vi "Super Market Billing System Edited.vi"() -> ()   [LabVIEW 2021]
uses:
  <vilib>/Utility/file.llb/Write Delimited Spreadsheet (string).vi
  <vilib>/regexp/Match Regular Expression.xnode
panel:
  in  "Tab Control":enum32{"Page 1", "Page 2", "Page 3"}(tab)
  out "Horizontal Progress Bar":u8(slide) scale=0.0..100.0
  in  "Password":string
  in  "Cashier User Name":string
  in  "OK Button":bool
  in  "Rise 5Kg":bool
  in  "Dal 1Kg":bool
  in  "Salt 400g":bool
  in  "Coconut Oil 1L":bool
  in  "Cilli Powder 100g":bool
  in  "Curry Powder 100g":bool
  in  "Turmeric Powder 50g":bool
  in  "Milk Powder 1kg":bool
  in  "Sugar  1kg":bool
  out "Rs.":dbl
  out "Rs.":dbl
  out "Rs.":dbl
  out "Rs.":dbl
  in  "Quantitiy":dbl min=0.0 format="%#.1f"
  out "Rs.":dbl
  in  "Quantitiy":dbl min=0.0 format="%#.1f"
  out "Rs":dbl
  in  "Quantitiy":dbl min=0.0 format="%#.1f"
  out "Rs.":dbl
  in  "Quantitiy":dbl min=0.0 format="%#.1f"
  in  "Quantitiy":dbl min=0.0 format="%#.1f"
  in  "Quantitiy":dbl min=0.0 format="%#.1f"
  in  "Quantitiy":dbl min=0.0 format="%#.1f"
  in  "Quantitiy":dbl min=0.0 format="%#.1f"
  in  "Tea 100g":bool
  in  "Quantitiy":dbl min=0.0 format="%#.1f"
  in  "Quantitiy":dbl min=0.0 format="%#.1f"
  out "Rs.":dbl
  out "Rs.":dbl
  out "Rs.":dbl
  out "Rs.":dbl
  out "Rs.":dbl
  out "Rs.":dbl
  out "Rs.":dbl
  out "Rs. 5":dbl
  out "Rs. 6":dbl
  out "Rs.":dbl
  out "Rs.":dbl
  out "Rs.":dbl
  out "Rs.":dbl
  out "Discount   Rs.":dbl format="%#.2f"
  in  "kg":dbl min=0.0 format="%#.3f"
  in  "Papaya":bool
  in  "kg":dbl min=0.0 format="%#.3f"
  in  "Graps":bool
  in  "kg":dbl min=0.0 format="%#.3f"
  in  "Orange":bool
  in  "kg":dbl min=0.0 format="%#.3f"
  in  "Apple":bool
  in  "kg":dbl min=0.0 format="%#.3f"
  in  "Banana":bool
  out "Bill   Rs.":dbl format="%#.2f"
  out "Discount percentage":string
  out "Total Bill   Rs.":dbl format="%#.2f"
  in  "kg":dbl min=0.0 format="%#.3f"
  in  "Cabege":bool
  in  "kg":dbl min=0.0 format="%#.3f"
  in  "Bringle":bool
  in  "kg":dbl min=0.0 format="%#.3f"
  in  "Beans":bool
  in  "kg":dbl min=0.0 format="%#.3f"
  in  "Leeks":bool
  in  "kg":dbl min=0.0 format="%#.3f"
  in  "Carrot":bool
  in  "stop":bool
  in  "stop 2":bool
  out "Bill Details":string
  in  "stop 3":bool
  # "WELCOME   TO  ABC                  SUPERMARCKET.."
  # "Price per 1kg (Rs.)"
  # "Quantities(kg)"
  # "Price  (Rs.)"
  # "Quantities"
  # "Fruits"
  # "Product List"
  # "Vegetables"
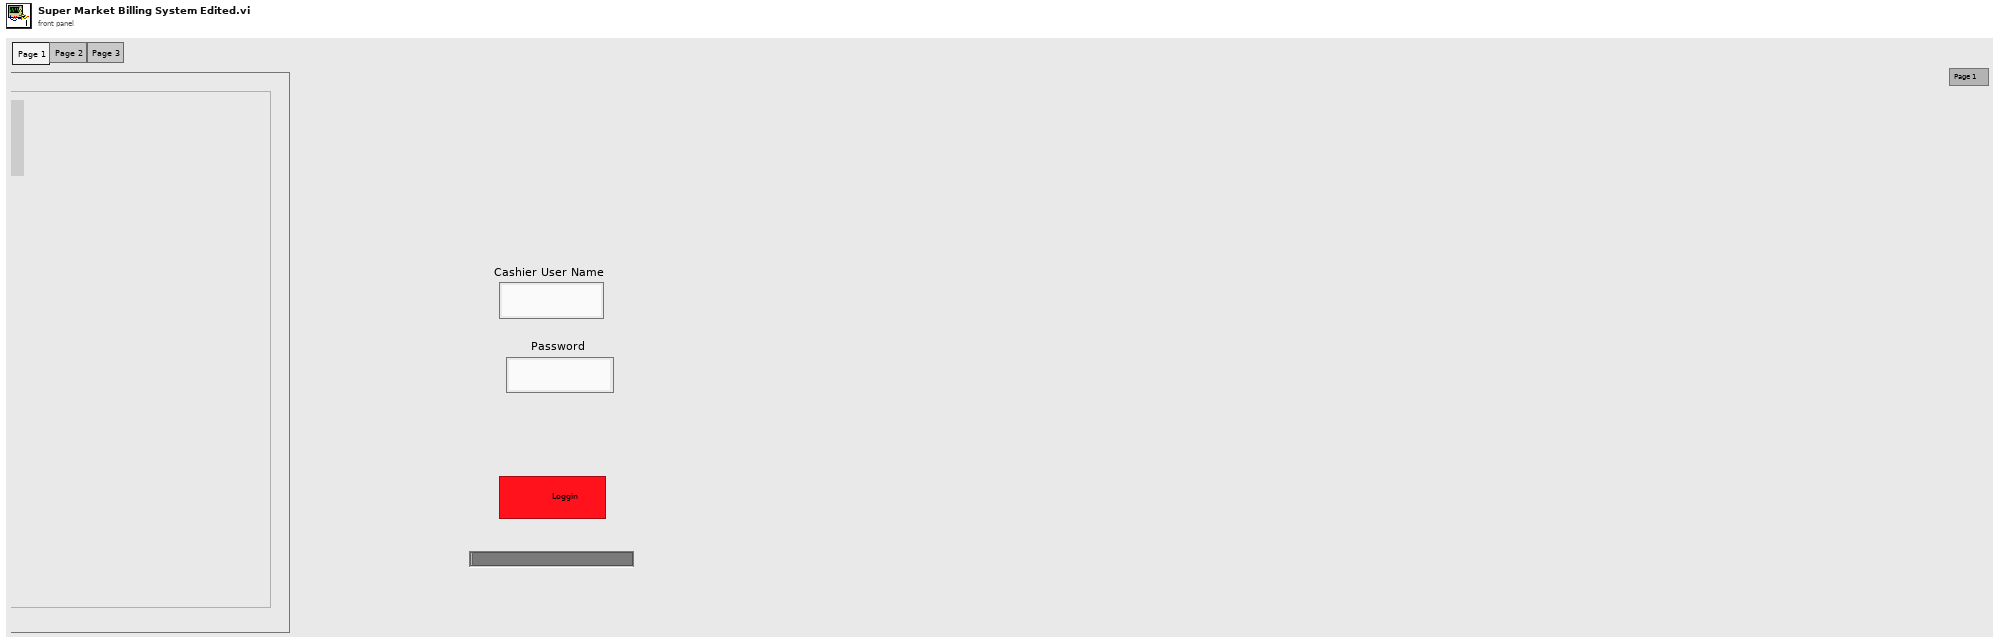
[diagram p1: front panel]
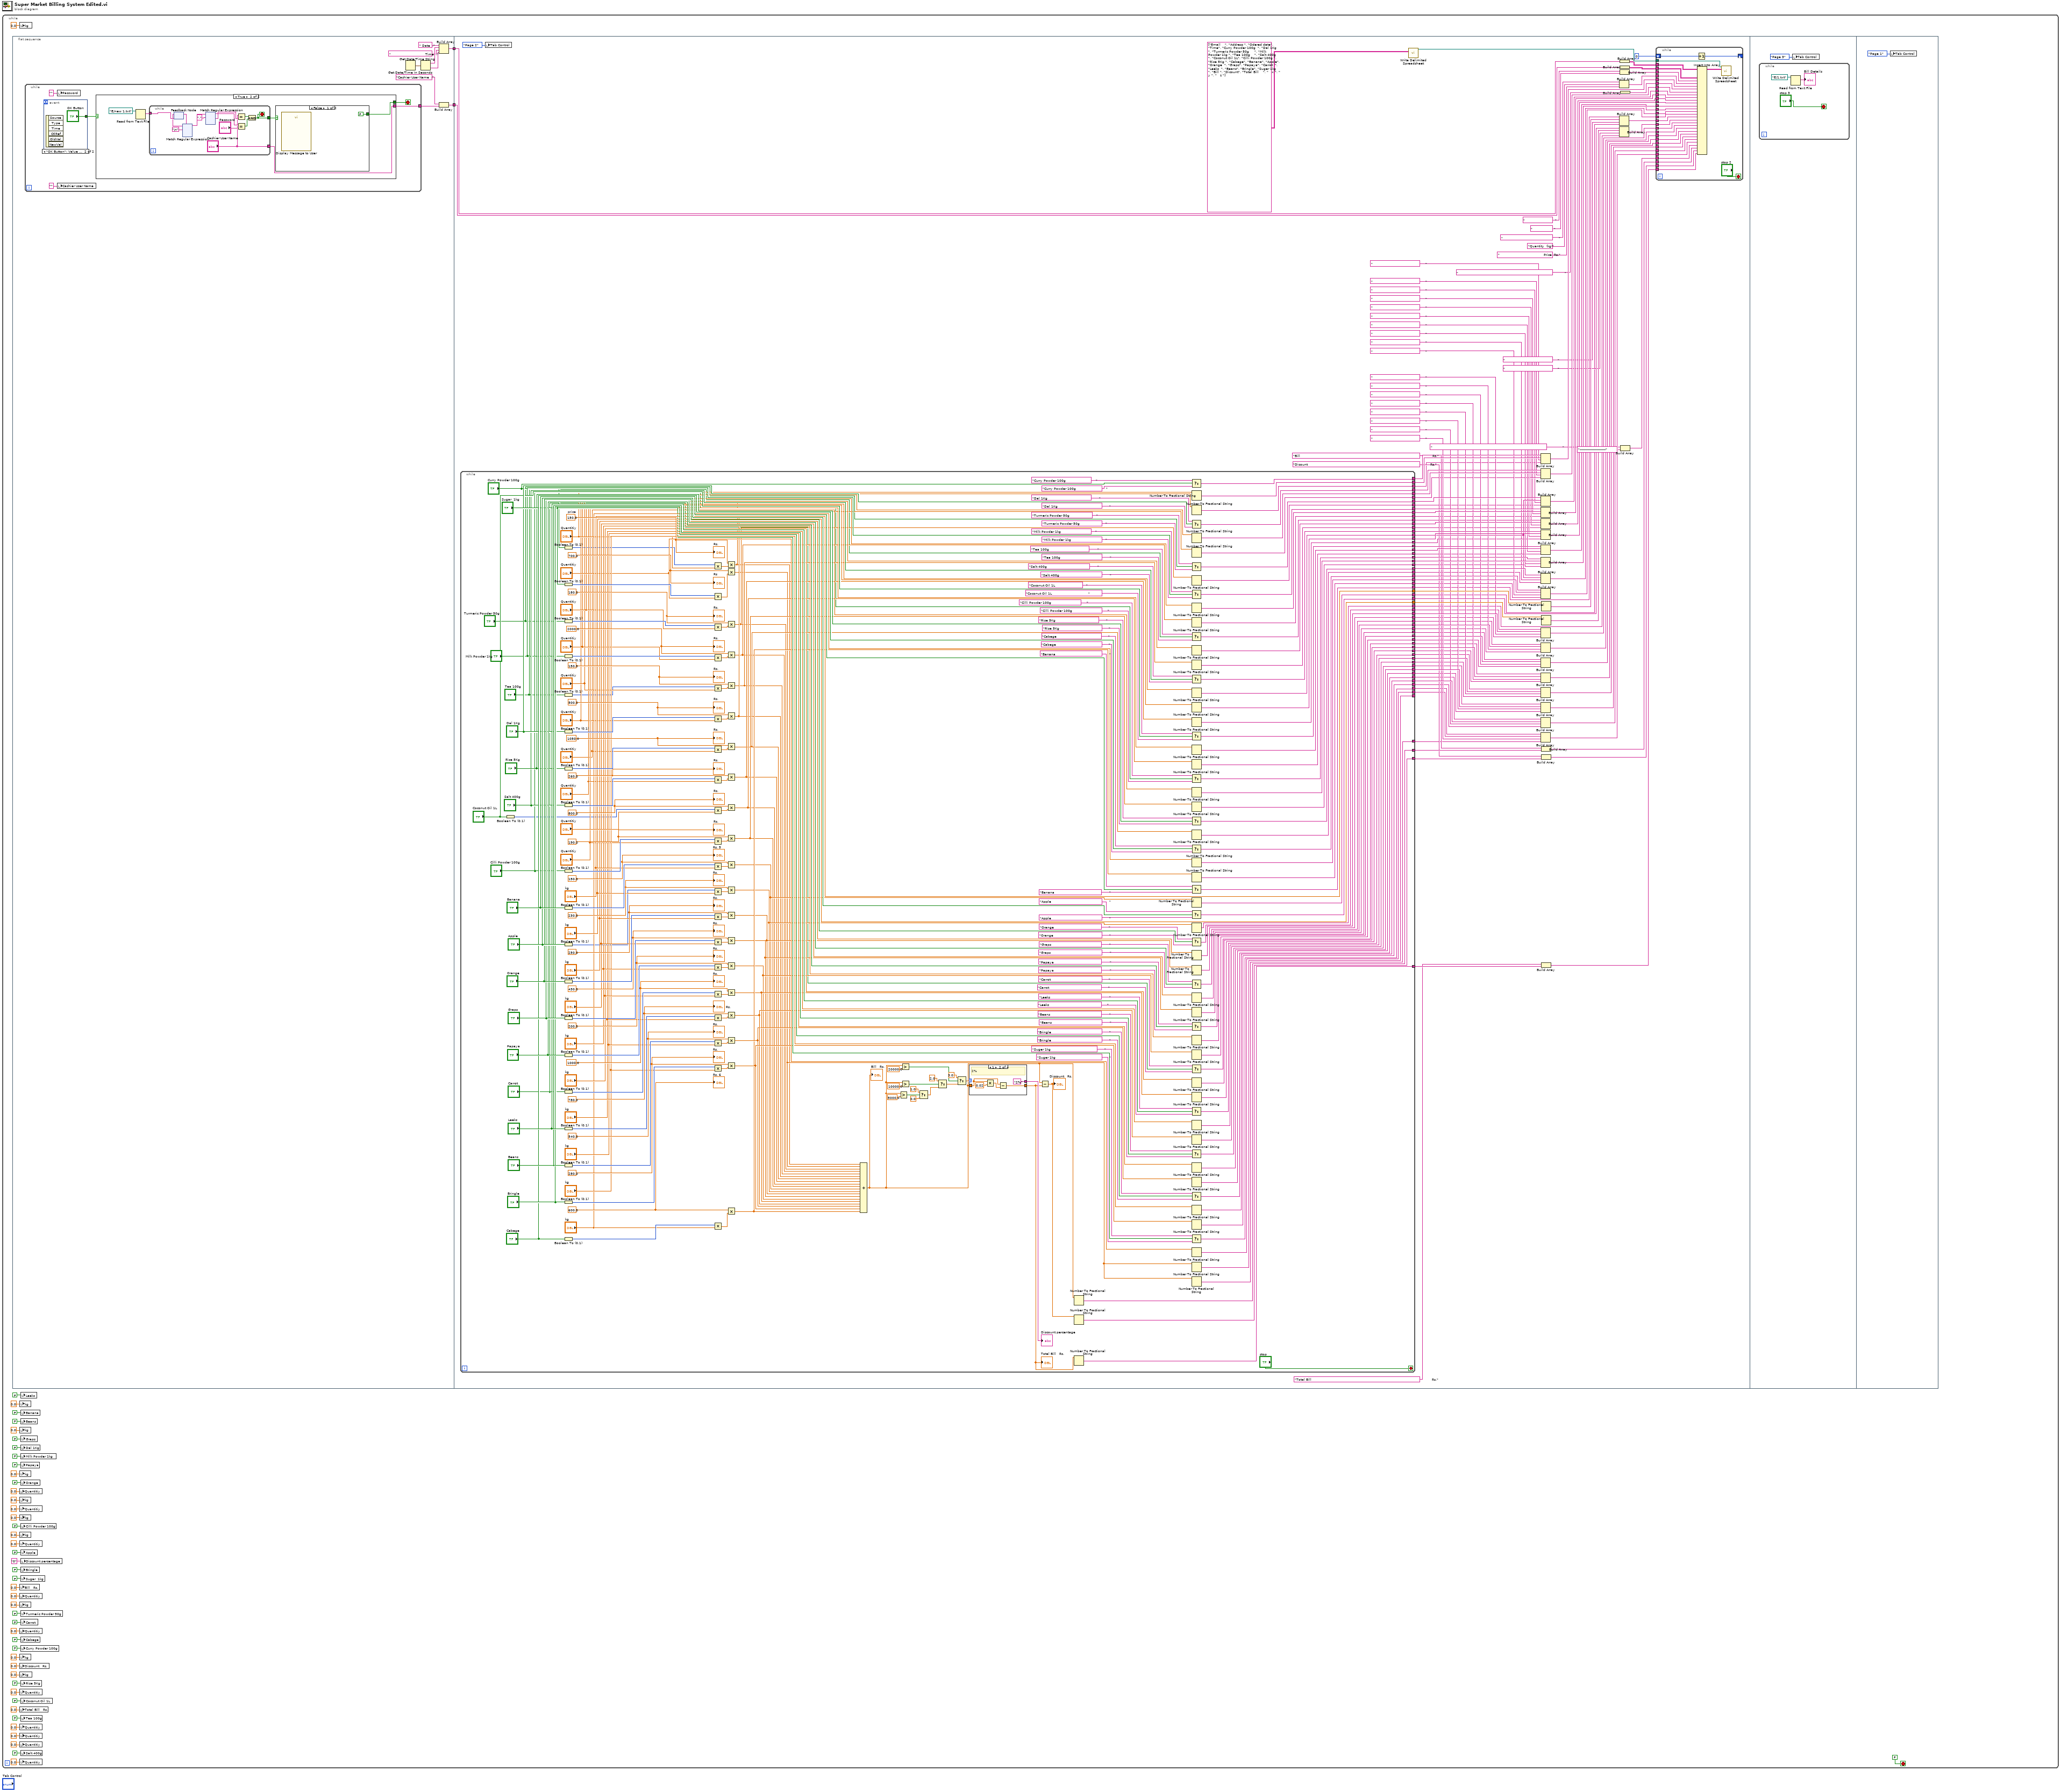
[diagram p0: block diagram]
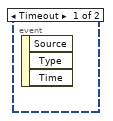
[diagram p2: hidden frame]
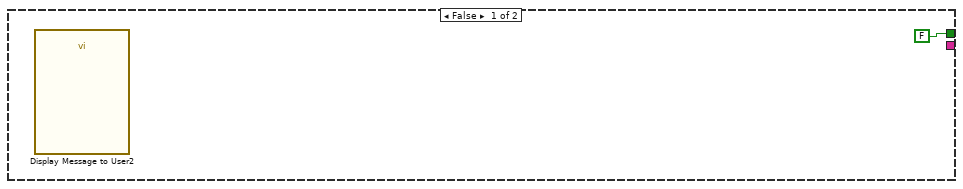
[diagram p3: hidden frame]
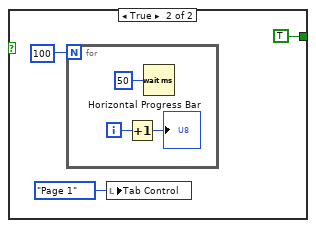
[diagram p4: hidden frame]
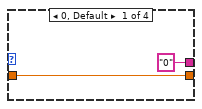
[diagram p5: hidden frame]
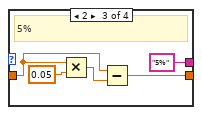
[diagram p6: hidden frame]
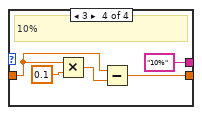
[diagram p7: hidden frame]
diagram:
  n1 = while {
    stop <- FALSE stop-if-true
    n2 = flat-sequence {
      tunnel: [w54] -> w46
      tunnel: [w50] -> w2
      tunnel: w46 -> [w452]
      tunnel: w2 -> [w390]
      frame #0 {
        n3 = while {
          tunnel: [w61] -> w48
          stop <- w60 stop-if-true
          n4 = event shown="[1] \"OK Button\": Value Change" {
            selector: _ -> [_ _]
            dyn-events: _ -> [_ _]
            timeout: _ -> [_ _]
            tunnel: [_ "OK Button"] -> w57
            event Timeout {
              n5 = event-data() -> ()  [unwired: 1 in, 3 out]
            }
            event "OK Button": Value Change {
              n6 = event-data() -> ()  [unwired: 1 in, 6 out]
            }
          }
          n7 = local write "Password"("" ("String 2")) -> ()
          n8 = local write "Cashier User Name"("" ("String")) -> ()
          n9 = case shown="True" w57 {
            tunnel: [_ w66] -> w61
            tunnel: [FALSE w65] -> w60
            frame False {
              n10 = call "Display Message to User2"() -> ()  [unwired: 10 in, 2 out]
            }
            frame True {
              n11 = Read from Text File(file (use dialog)=path "E:/new 1.txt") -> (text=w68:string)  [unwired: 3 in, 3 out]
              n12 = while {
                tunnel: w68 -> [w88]
                tunnel: ["Cashier User Name"] -> w66
                tunnel: [w76] -> w64
                stop <- w76 stop-if-true
                n13 = feedback #1(w88) -> (w87:string)
                n14 = xnode "Match Regular Expression"("input string"=w87, "regular expression"="\n") -> ("before match"=w84:string, "after match"=w86:string)  [unwired: 4 in, 3 out]
                n15 = feedback-in #1(w86) -> ()
                n16 = xnode "Match Regular Expression"("input string"=w84, "regular expression"=",") -> ("before match"=w81:string, "after match"=w82:string)  [unwired: 4 in, 3 out]
                n17 = Equal?(x="Cashier User Name", y=w81) -> (x = y?=w79:bool)
                n18 = Equal?(x=w82, y="Password") -> (x = y?=w78:bool)
                n19 = And(x=w79, y=w78) -> (x .and. y?=w76:bool)
              }
              n20 = case shown="False" w64 {
                tunnel: [FALSE TRUE] -> w65
                frame False {
                  n21 = call "Display Message to User"() -> ()  [unwired: 10 in, 2 out]
                }
                frame True {
                  n22 = for {
                    N: 100 -> [_]
                    i -> [w73]
                    n23 = Increment(x=w73) -> (x+1=→"Horizontal Progress Bar":i32)
                    n24 = Wait (ms)(milliseconds to wait=u32 50 ("millisecond timer value")) -> ()  [unwired: 1 out]
                  }
                  n25 = local write "Tab Control"(enum32{"Page 1", "Page 2"}."Page 1" ("Tab Control")) -> ()
                }
              }
            }
          }
        }
        n26 = Get Date/Time In Seconds() -> (seconds since 1Jan1904=w55:timestamp)
        n27 = Get Date/Time String(seconds (now)=w55) -> (date string=w53:string, time string=w56:string)  [unwired: 2 in]
        n28 = Build Array(" Date  :" ("element"), w53, "                                Time  :" ("element"), w56) -> (w54:string[])
        n29 = Build Array("Cashier User Name  :" ("element"), w48) -> (w50:string[])
      }
      frame #1 {
        n30 = while {
          tunnel: [w658] -> w444
          tunnel: [w655] -> w446
          tunnel: [w654] -> w447
          tunnel: [w646] -> w358
          tunnel: [w626] -> w413
          tunnel: [w625] -> w331
          tunnel: [w617] -> w327
          tunnel: [w616] -> w326
          tunnel: [w615] -> w325
          tunnel: [w614] -> w324
          tunnel: [w613] -> w328
          tunnel: [w612] -> w329
          tunnel: [w611] -> w404
          tunnel: ["kg"] -> w451
          tunnel: ["kg"] -> w450
          tunnel: [w607] -> w411
          tunnel: [w605] -> w410
          tunnel: [w602] -> w409
          tunnel: [w601] -> w408
          tunnel: [w600] -> w407
          tunnel: [w597] -> w406
          tunnel: [w594] -> w405
          tunnel: [w593] -> w403
          tunnel: [w565] -> w330
          tunnel: [w564] -> w443
          tunnel: [w563] -> w441
          tunnel: [w562] -> w440
          tunnel: [w561] -> w345
          tunnel: [w560] -> w437
          tunnel: [w559] -> w430
          tunnel: [w558] -> w434
          tunnel: [w557] -> w432
          tunnel: [w487] -> w431
          tunnel: [w554] -> w442
          tunnel: [w538] -> w378
          tunnel: [w552] -> w428
          tunnel: [w550] -> w439
          tunnel: [w548] -> w438
          tunnel: [w543] -> w436
          tunnel: [w542] -> w435
          tunnel: [w541] -> w433
          tunnel: [w540] -> w429
          tunnel: [w537] -> w377
          tunnel: [w536] -> w375
          tunnel: [w515] -> w373
          tunnel: [w514] -> w371
          tunnel: [w513] -> w369
          tunnel: [w511] -> w367
          tunnel: [w510] -> w365
          tunnel: [w499] -> w363
          tunnel: [w509] -> w361
          tunnel: [w508] -> w359
          tunnel: [w498] -> w356
          tunnel: [w507] -> w354
          tunnel: [w506] -> w351
          tunnel: [w505] -> w350
          tunnel: [w494] -> w348
          tunnel: [w504] -> w346
          tunnel: [w493] -> w343
          tunnel: [w503] -> w341
          tunnel: [w502] -> w339
          tunnel: [w501] -> w337
          tunnel: [w500] -> _
          stop <- "stop" stop-if-true
          w670 = 200.0 ("price")
          w667 = 430.0 ("price")
          w664 = 250.0 ("price")
          w662 = 230.0 ("price")
          w659 = 150.0 ("price")
          w685 = 600.0 ("price")
          w682 = 280.0 ("price")
          w679 = 540.0 ("price")
          w676 = 780.0 ("price")
          w673 = 1000.0 ("price")
          w712 = 150.0 ("price")
          w710 = 700.0 ("price")
          w707 = 2000.0 ("price")
          w704 = 180.0 ("price")
          w701 = 150.0  # price
          w724 = 190.0 ("price")
          w722 = 800.0 ("price")
          w719 = 260.0 ("price")
          w717 = 500.0 ("price")
          w714 = 1050.0 ("price")
          n31 = Boolean To (0,1)(Boolean="Coconut Oil 1L") -> (0, 1=w495:i16)
          n32 = Boolean To (0,1)(Boolean="Curry Powder 100g") -> (0, 1=w488:i16)
          n33 = Boolean To (0,1)(Boolean="Sugar  1kg") -> (0, 1=w711:i16)
          n34 = Boolean To (0,1)(Boolean="Turmeric Powder 50g") -> (0, 1=w705:i16)
          n35 = Boolean To (0,1)(Boolean="Milk Powder 1kg") -> (0, 1=w706:i16)
          n36 = Boolean To (0,1)(Boolean="Tea 100g") -> (0, 1=w491:i16)
          n37 = Boolean To (0,1)(Boolean="Dal 1Kg") -> (0, 1=w651:i16)
          n38 = Boolean To (0,1)(Boolean="Rise 5Kg") -> (0, 1=w653:i16)
          n39 = Boolean To (0,1)(Boolean="Salt 400g") -> (0, 1=w718:i16)
          n40 = Boolean To (0,1)(Boolean="Cilli Powder 100g") -> (0, 1=w652:i16)
          n41 = Boolean To (0,1)(Boolean="Banana") -> (0, 1=w650:i16)
          n42 = Boolean To (0,1)(Boolean="Apple") -> (0, 1=w497:i16)
          n43 = Boolean To (0,1)(Boolean="Orange") -> (0, 1=w663:i16)
          n44 = Boolean To (0,1)(Boolean="Graps") -> (0, 1=w668:i16)
          n45 = Boolean To (0,1)(Boolean="Papaya") -> (0, 1=w669:i16)
          n46 = Boolean To (0,1)(Boolean="Carrot") -> (0, 1=w672:i16)
          n47 = Boolean To (0,1)(Boolean="Leeks") -> (0, 1=w677:i16)
          n48 = Boolean To (0,1)(Boolean="Beans") -> (0, 1=w678:i16)
          n49 = Boolean To (0,1)(Boolean="Bringle") -> (0, 1=w683:i16)
          n50 = Boolean To (0,1)(Boolean="Cabege") -> (0, 1=w684:i16)
          n51 = Multiply(x=w488, y="Quantitiy") -> (x*y=w702:dbl)
          n52 = Multiply(x=w711, y="Quantitiy") -> (x*y=w709:dbl)
          n53 = Multiply(x=w705, y="Quantitiy") -> (x*y=w703:dbl)
          n54 = Multiply(x=w706, y="Quantitiy") -> (x*y=w708:dbl)
          n55 = Multiply(x=w491, y="Quantitiy") -> (x*y=w713:dbl)
          n56 = Multiply(x=w651, y="Quantitiy") -> (x*y=w716:dbl)
          n57 = Multiply(x=w653, y="Quantitiy") -> (x*y=w715:dbl)
          n58 = Multiply(x=w718, y="Quantitiy") -> (x*y=w720:dbl)
          n59 = Multiply(x=w495, y="Quantitiy") -> (x*y=w721:dbl)
          n60 = Multiply(x=w652, y="Quantitiy") -> (x*y=w725:dbl)
          n61 = Multiply(x=w650, y="kg") -> (x*y=w660:dbl)
          n62 = Multiply(x=w497, y="kg") -> (x*y=w661:dbl)
          n63 = Multiply(x=w663, y="kg") -> (x*y=w665:dbl)
          n64 = Multiply(x=w668, y="kg") -> (x*y=w666:dbl)
          n65 = Multiply(x=w669, y="kg") -> (x*y=w671:dbl)
          n66 = Multiply(x=w672, y="kg") -> (x*y=w674:dbl)
          n67 = Multiply(x=w677, y="kg") -> (x*y=w675:dbl)
          n68 = Multiply(x=w678, y="kg") -> (x*y=w680:dbl)
          n69 = Multiply(x=w683, y="kg") -> (x*y=w681:dbl)
          n70 = Multiply(x=w684, y="kg") -> (x*y=w686:dbl)
          n71 = Multiply(x=w701, y=w702) -> (x*y=w489:dbl)
          n72 = Multiply(x=w710, y=w709) -> (x*y=w516:dbl)
          n73 = Multiply(x=w704, y=w703) -> (x*y=w518:dbl)
          n74 = Multiply(x=w707, y=w708) -> (x*y=w519:dbl)
          n75 = Multiply(x=w712, y=w713) -> (x*y=w520:dbl)
          n76 = Multiply(x=w717, y=w716) -> (x*y=w522:dbl)
          n77 = Multiply(x=w714, y=w715) -> (x*y=w521:dbl)
          n78 = Multiply(x=w719, y=w720) -> (x*y=w523:dbl)
          n79 = Multiply(x=w722, y=w721) -> (x*y=w524:dbl)
          n80 = Multiply(x=w724, y=w725) -> (x*y=w525:dbl)
          n81 = Multiply(x=w659, y=w660) -> (x*y=w526:dbl)
          n82 = Multiply(x=w662, y=w661) -> (x*y=w527:dbl)
          n83 = Multiply(x=w664, y=w665) -> (x*y=w528:dbl)
          n84 = Multiply(x=w667, y=w666) -> (x*y=w529:dbl)
          n85 = Multiply(x=w670, y=w671) -> (x*y=w530:dbl)
          n86 = Multiply(x=w673, y=w674) -> (x*y=w531:dbl)
          n87 = Multiply(x=w676, y=w675) -> (x*y=w534:dbl)
          n88 = Multiply(x=w679, y=w680) -> (x*y=w533:dbl)
          n89 = Multiply(x=w682, y=w681) -> (x*y=w535:dbl)
          n90 = Multiply(x=w685, y=w686) -> (x*y=w532:dbl)
          n91 = Compound Arithmetic op=ADD(w489, w516, w518, w519, w520, w522, w521, w523, w524, w525, w526, w527, w528, w529, w530, w531, w534, w533, w535, w532) -> (w517:dbl)
          "Bill   Rs." <- w517
          n92 = Greater?(x=w517, y=5000.0) -> (0:w698:bool)
          n93 = Greater?(x=w517, y=20000.0) -> (0:w700:bool)
          n94 = Greater?(x=w517, y=10000.0) -> (0:w699:bool)
          n95 = Select(t=1.0, s=w698, f=0.0) -> (s? t:f=w694:dbl)
          n96 = Select(t=2.0, s=w699, f=w694) -> (s? t:f=w695:dbl)
          n97 = Select(t=3.0, s=w700, f=w695) -> (s? t:f=w696:dbl)
          n98 = case shown="1" w696 {
            tunnel: [w727 w731 w734 w739] -> w657
            tunnel: w517 -> [w727 w730 w735 w740]
            tunnel: ["0" ("discount") "2%" ("discount") "5%" ("discount") "10%" ("discount")] -> w697
            frame 0, Default {
            }
            frame 1 {
              # "2%"
              n99 = Multiply(x=w730, y=0.02) -> (x*y=w728:dbl)
              n100 = Subtract(x=w730, y=w728) -> (x-y=w731:dbl)
            }
            frame 2 {
              # "5%"
              n101 = Multiply(x=w735, y=0.05) -> (x*y=w736:dbl)
              n102 = Subtract(x=w735, y=w736) -> (x-y=w734:dbl)
            }
            frame 3 {
              # "10%"
              n103 = Multiply(x=w740, y=0.1) -> (x*y=w741:dbl)
              n104 = Subtract(x=w740, y=w741) -> (x-y=w739:dbl)
            }
          }
          "Total Bill   Rs." <- w657
          "Discount percentage" <- w697
          n105 = Subtract(x=w517, y=w657) -> (x-y=w656:dbl)
          "Discount   Rs." <- w656
          n106 = Number To Fractional String(number=w517) -> (F-format string=w658:string)  [unwired: 3 in]
          n107 = Number To Fractional String(number=w656) -> (F-format string=w654:string)  [unwired: 3 in]
          n108 = Number To Fractional String(number=w657) -> (F-format string=w655:string)  [unwired: 3 in]
          n109 = Select(t="Curry Powder 100g                            ", s="Curry Powder 100g", f="Curry Powder 100g                            ") -> (s? t:f=w564:string)
          n110 = Number To Fractional String(number="Quantitiy") -> (F-format string=w554:string)  [unwired: 3 in]
          n111 = Number To Fractional String(number=w489) -> (F-format string=w501:string)  [unwired: 3 in]
          n112 = Select(t="Dal 1Kg                                                ", s="Dal 1Kg", f="Dal 1Kg                                                ") -> (s? t:f=w487:string)
          n113 = Number To Fractional String(number="Quantitiy") -> (F-format string=w540:string)  [unwired: 3 in]
          n114 = Number To Fractional String(number=w522) -> (F-format string=w494:string)  [unwired: 3 in]
          n115 = Select(t="Turmeric Powder 50g                         ", s="Turmeric Powder 50g", f="Turmeric Powder 50g                        ") -> (s? t:f=w563:string)
          n116 = Number To Fractional String(number=w518) -> (F-format string=w502:string)  [unwired: 3 in]
          n117 = Select(t="Milk Powder 1kg                                ", s="Milk Powder 1kg", f="Milk Powder 1kg                                ") -> (s? t:f=w562:string)
          n118 = Number To Fractional String(number="Quantitiy") -> (F-format string=w550:string)  [unwired: 3 in]
          n119 = Number To Fractional String(number=w519) -> (F-format string=w503:string)  [unwired: 3 in]
          n120 = Select(t="Tea 100g                                             ", s="Tea 100g", f="Tea 100g                                              ") -> (s? t:f=w561:string)
          n121 = Number To Fractional String(number="Quantitiy") -> (F-format string=w548:string)  [unwired: 3 in]
          n122 = Number To Fractional String(number=w520) -> (F-format string=w493:string)  [unwired: 3 in]
          n123 = Select(t="Salt 400g                                               ", s="Salt 400g", f="Salt 400g                                               ") -> (s? t:f=w560:string)
          n124 = Number To Fractional String(number="Quantitiy") -> (F-format string=w552:string)  [unwired: 3 in]
          n125 = Number To Fractional String(number="Quantitiy") -> (F-format string=w543:string)  [unwired: 3 in]
          n126 = Number To Fractional String(number=w523) -> (F-format string=w505:string)  [unwired: 3 in]
          n127 = Select(t="Coconut Oil 1L                             ", s="Coconut Oil 1L", f="Coconut Oil 1L                                  ") -> (s? t:f=w559:string)
          n128 = Number To Fractional String(number="Quantitiy") -> (F-format string=w542:string)  [unwired: 3 in]
          n129 = Number To Fractional String(number=w524) -> (F-format string=w506:string)  [unwired: 3 in]
          n130 = Select(t="Cilli Powder 100g                                 ", s="Cilli Powder 100g", f="Cilli Powder 100g                                 ") -> (s? t:f=w558:string)
          n131 = Number To Fractional String(number="Quantitiy") -> (F-format string=w541:string)  [unwired: 3 in]
          n132 = Number To Fractional String(number=w525) -> (F-format string=w507:string)  [unwired: 3 in]
          n133 = Select(t="Rise 5Kg                                               ", s="Rise 5Kg", f="Rise 5Kg                                              ") -> (s? t:f=w557:string)
          n134 = Number To Fractional String(number=w521) -> (F-format string=w504:string)  [unwired: 3 in]
          n135 = Select(t="Cabege                                                ", s="Cabege", f="Cabege                                                 ") -> (s? t:f=w611:string)
          n136 = Number To Fractional String(number="kg") -> (F-format string=w593:string)  [unwired: 3 in]
          n137 = Number To Fractional String(number=w532) -> (F-format string=w515:string)  [unwired: 3 in]
          n138 = Select(t="Banana                                                  ", s="Banana", f="Banana                                                   ") -> (s? t:f=w646:string)
          n139 = Number To Fractional String(number=w526) -> (F-format string=w498:string)  [unwired: 3 in]
          n140 = Select(t="Apple                                                      ", s="Apple", f="Apple                                                      ") -> (s? t:f=w626:string)
          n141 = Number To Fractional String(number=w527) -> (F-format string=w508:string)  [unwired: 3 in]
          n142 = Select(t="Orange                                                   ", s="Orange", f="Orange                                                    ") -> (s? t:f=w625:string)
          n143 = Number To Fractional String(number="kg") -> (F-format string=w607:string)  [unwired: 3 in]
          n144 = Number To Fractional String(number=w528) -> (F-format string=w509:string)  [unwired: 3 in]
          n145 = Select(t="Graps                                                      " ("f"), s="Graps", f="Graps                                                       ") -> (s? t:f=w617:string)
          n146 = Number To Fractional String(number="kg") -> (F-format string=w605:string)  [unwired: 3 in]
          n147 = Number To Fractional String(number=w529) -> (F-format string=w499:string)  [unwired: 3 in]
          n148 = Select(t="Papaya                                                    ", s="Papaya", f="Papaya                                                    ") -> (s? t:f=w616:string)
          n149 = Number To Fractional String(number="kg") -> (F-format string=w602:string)  [unwired: 3 in]
          n150 = Number To Fractional String(number=w530) -> (F-format string=w510:string)  [unwired: 3 in]
          n151 = Select(t="Carrot                                                      ", s="Carrot", f="Carrot                                                       ") -> (s? t:f=w615:string)
          n152 = Number To Fractional String(number="kg") -> (F-format string=w601:string)  [unwired: 3 in]
          n153 = Number To Fractional String(number=w531) -> (F-format string=w511:string)  [unwired: 3 in]
          n154 = Select(t="Leeks                                                       ", s="Leeks", f="Leeks                                                      ") -> (s? t:f=w614:string)
          n155 = Number To Fractional String(number="kg") -> (F-format string=w600:string)  [unwired: 3 in]
          n156 = Number To Fractional String(number=w534) -> (F-format string=w513:string)  [unwired: 3 in]
          n157 = Select(t="Beans                                                       ", s="Beans", f="Beans                                                      ") -> (s? t:f=w613:string)
          n158 = Number To Fractional String(number="kg") -> (F-format string=w597:string)  [unwired: 3 in]
          n159 = Number To Fractional String(number=w533) -> (F-format string=w514:string)  [unwired: 3 in]
          n160 = Select(t="Bringle                                                      ", s="Bringle", f="Bringle                                                      ") -> (s? t:f=w612:string)
          n161 = Number To Fractional String(number="kg") -> (F-format string=w594:string)  [unwired: 3 in]
          n162 = Number To Fractional String(number=w535) -> (F-format string=w536:string)  [unwired: 3 in]
          n163 = Select(t="Suger 1kg                                                  ", s="Sugar  1kg", f="Suger 1kg                                                  ") -> (s? t:f=w565:string)
          n164 = Number To Fractional String(number="Quantitiy") -> (F-format string=w538:string)  [unwired: 3 in]
          n165 = Number To Fractional String(number=w516) -> (F-format string=w500:string)  [unwired: 3 in]
          n166 = Number To Fractional String(number=w516) -> (F-format string=w537:string)  [unwired: 3 in]
          "Rs." <- w714
          "Rs." <- w717
          "Rs." <- w719
          "Rs." <- w722
          "Rs." <- w724
          "Rs." <- w701
          "Rs." <- w704
          "Rs." <- w707
          "Rs" <- w710
          "Rs." <- w712
          "Rs." <- w673
          "Rs." <- w676
          "Rs." <- w679
          "Rs." <- w682
          "Rs. 6" <- w685
          "Rs. 5" <- w659
          "Rs." <- w662
          "Rs." <- w664
          "Rs." <- w667
          "Rs." <- w670
        }
        n167 = local write "Tab Control"(enum32{"Page 1", "Page 2"}."Page 2" ("Tab Control")) -> ()
        n168 = call-poly <vilib>:"Write Delimited Spreadsheet.vi"("2D data"=string[][] [["Email    "], ["Address "], ["Odered date"], ["Time"], ["Curry Powder 100g  "], ["Dal 1Kg   "], ["Turmeric Powder 50g     "], ["Milk Powder 1kg "], ["Tea 100g    "], ["Salt 400g   "], ["Coconut Oil 1L"], ["Cilli Powder 100g "], ["Rise 5Kg "], ["Cabege"], ["Banana"], ["Apple"], ["Orange  "], ["Graps"], ["Papaya"], ["Carrot  "], ["Leeks  "], ["Beans"], ["Bringle"], ["Suger 1kg  "], ["Bill "], ["Dicount"], ["Total Bill    "], ["   x "], ["   y "], ["   z "]] ("delimiter (\\t)")) -> ("new file path (Not A Path if cancelled)"=w448:path)  [unwired: 13 in, 1 out]
        n169 = Build Array(w443, w442, "                                                 " ("element"), w337) -> (w423:string[])
        n170 = Build Array(w431, w429, "                                                 " ("element"), w348) -> (w415:string[])
        n171 = Build Array(w441, w428, "                                                 " ("element"), w339) -> (w422:string[])
        n172 = Build Array(w440, w439, "                                                 " ("element"), w341) -> (w421:string[])
        n173 = Build Array(w345, w438, "                                                 " ("element"), w343) -> (w420:string[])
        n174 = Build Array(w437, w436, "                                                 " ("element"), w350) -> (w419:string[])
        n175 = Build Array(w430, w435, "                                                 " ("element"), w351) -> (w418:string[])
        n176 = Build Array(w434, w433, "                                                 " ("element"), w354) -> (w417:string[])
        n177 = Build Array(w432, w428, "                                                 " ("element"), w346) -> (w416:string[])
        n178 = Build Array(w404, w403, "                                                 " ("element"), w373) -> (w393:string[])
        n179 = Build Array(w331, w411, "                                                 " ("element"), w361) -> (w400:string[])
        n180 = Build Array(w327, w410, "                                                 " ("element"), w363) -> (w399:string[])
        n181 = Build Array(w326, w409, "                                                 " ("element"), w365) -> (w398:string[])
        n182 = Build Array(w325, w408, "                                                 " ("element"), w367) -> (w397:string[])
        n183 = Build Array(w324, w407, "                                                 " ("element"), w369) -> (w396:string[])
        n184 = Build Array(w328, w406, "                                                 " ("element"), w371) -> (w395:string[])
        n185 = Build Array(w329, w405, "                                                 " ("element"), w375) -> (w394:string[])
        n186 = Build Array(w330, w378, "                                                 " ("element"), w377) -> (w424:string[])
        n187 = Build Array("Bill                                                                                                                           Rs." ("element"), w444) -> (w426:string[])
        n188 = Build Array("Dicount                                                                                                                  Rs." ("element"), w447) -> (w380:string[])
        n189 = Build Array("Total Bill                                                                                                                Rs." ("element"), w446) -> (w425:string[])
        n190 = Number To Fractional String(number=w451) -> (F-format string=w414:string)  [unwired: 3 in]
        n191 = Number To Fractional String(number=w450) -> (F-format string=w412:string)  [unwired: 3 in]
        n192 = Build Array(w358, w414, "                                                 " ("element"), w356) -> (w402:string[])
        n193 = Build Array(w413, w412, "                                                 " ("element"), w359) -> (w401:string[])
        n194 = Build Array("                                                    " ("element"), "Quantity  (kg)" ("element"), "                                         Price  Rs." ("element")) -> (w382:string[])
        n195 = Build Array(w452) -> (w427:string[][])
        n196 = Build Array(w390) -> (w389:string[][])
        n197 = Build Array("                            ", "                    " ("element")) -> (w385:string[])
        n198 = Build Array("                                                                                                   ") -> (w332:string[])
        n199 = Build Array("                                                                                                                         ", "------------------------" ("element")) -> (w335:string[])
        n200 = while {
          tunnel: w448 -> [w486]
          shift-right: [w483] -> _
          shift-left: 0 -> [w484]
          tunnel: w427 -> [w482]
          tunnel: w426 -> [w455]
          tunnel: w380 -> [w454]
          tunnel: w425 -> [w453]
          tunnel: w424 -> [w458]
          tunnel: w423 -> [w461]
          tunnel: w422 -> [w463]
          tunnel: w421 -> [w464]
          tunnel: w420 -> [w465]
          tunnel: w419 -> [w466]
          tunnel: w418 -> [w467]
          tunnel: w417 -> [w468]
          tunnel: w416 -> [w469]
          tunnel: w415 -> [w462]
          tunnel: w402 -> [w471]
          tunnel: w401 -> [w472]
          tunnel: w400 -> [w473]
          tunnel: w399 -> [w474]
          tunnel: w398 -> [w475]
          tunnel: w397 -> [w476]
          tunnel: w396 -> [w477]
          tunnel: w395 -> [w478]
          tunnel: w394 -> [w479]
          tunnel: w393 -> [w470]
          tunnel: w389 -> [w480]
          tunnel: w385 -> [w460]
          tunnel: w382 -> [w459]
          tunnel: w335 -> [w457]
          tunnel: w332 -> [w456]
          stop <- "stop 2" stop-if-true
          n201 = Increment(x=w484) -> (x+1=w483:i32)
          n202 = Insert Into Array "Insert Into Array"(array=w482, new element #1=w480, new element #2=w460, new element #3=w459, new element #4=w461, new element #5=w456, new element #6=w462, new element #7=w463, new element #8=w464, new element #9=w465, new element #10=w466, new element #11=w467, new element #12=w468, new element #13=w469, new element #14=w470, new element #15=w471, new element #16=w472, new element #17=w473, new element #18=w474, new element #19=w475, new element #20=w476, new element #21=w477, new element #22=w478, new element #23=w479, new element #24=w458, new element #25=w457, new element #26=w455, new element #27=w454, new element #28=w453) -> (w481:string[][])  [unwired: 2 in]
          n203 = call-poly <vilib>:"Write Delimited Spreadsheet.vi"("file path (dialog if empty)"=w486, "2D data"=w481) -> ()  [unwired: 12 in, 2 out]
        }
      }
      frame #2 {
        n204 = while {
          stop <- "stop 3" stop-if-true
          n205 = Read from Text File(file (use dialog)=path "E:/1.txt") -> (text=→"Bill Details":string)  [unwired: 3 in, 3 out]
        }
        n206 = local write "Tab Control"(enum32{"Page 1", "Page 2", "Page 3"}."Page 3" ("Tab Control")) -> ()
      }
      frame #3 {
        n207 = local write "Tab Control"(enum32{"Page 1", "Page 2"}."Page 1" ("Tab Control")) -> ()
      }
    }
    n208 = local write "kg"(0.0 ("kg")) -> ()
    n209 = local write "kg"(0.0 ("kg")) -> ()
    n210 = local write "kg"(0.0 ("kg")) -> ()
    n211 = local write "kg"(0.0 ("kg")) -> ()
    n212 = local write "Quantitiy"(0.0 ("Quantities")) -> ()
    n213 = local write "kg"(0.0 ("kg")) -> ()
    n214 = local write "Quantitiy"(0.0 ("quantity 15")) -> ()
    n215 = local write "kg"(0.0 ("kg")) -> ()
    n216 = local write "kg"(0.0 ("kg")) -> ()
    n217 = local write "Quantitiy"(0.0 ("quantity 17")) -> ()
    n218 = local write "Bill   Rs."(0.0 ("Bill   Rs.")) -> ()
    n219 = local write "Quantitiy"(0.0 ("quantity 10")) -> ()
    n220 = local write "kg"(0.0 ("kg")) -> ()
    n221 = local write "Quantitiy"(0.0 ("quantity 12")) -> ()
    n222 = local write "kg"(0.0 ("kg")) -> ()
    n223 = local write "Discount   Rs."(0.0 ("Discount   Rs.")) -> ()
    n224 = local write "kg"(0.0 ("kg")) -> ()
    n225 = local write "Quantitiy"(0.0 ("quantity 13")) -> ()
    n226 = local write "Total Bill   Rs."(0.0 ("Total Bill   Rs.")) -> ()
    n227 = local write "Quantitiy"(0.0 ("quantity 14")) -> ()
    n228 = local write "Quantitiy"(0.0 ("quantity 11")) -> ()
    n229 = local write "Quantitiy"(0.0 ("Quantities 4")) -> ()
    n230 = local write "Quantitiy"(0.0 ("quantity 16")) -> ()
    n231 = local write "Leeks"(FALSE ("Leeks")) -> ()
    n232 = local write "Banana"(FALSE ("Banana")) -> ()
    n233 = local write "Beans"(FALSE ("Beans")) -> ()
    n234 = local write "Graps"(FALSE ("Graps")) -> ()
    n235 = local write "Dal 1Kg"(FALSE ("Dal 1Kg")) -> ()
    n236 = local write "Milk Powder 1kg"(FALSE ("Milk Powder 1kg")) -> ()
    n237 = local write "Papaya"(FALSE ("Papaya")) -> ()
    n238 = local write "Orange"(FALSE ("Orange")) -> ()
    n239 = local write "Cilli Powder 100g"(FALSE ("Cilli Powder 100g")) -> ()
    n240 = local write "Apple"(FALSE ("Apple")) -> ()
    n241 = local write "Bringle"(FALSE ("Bringle")) -> ()
    n242 = local write "Sugar  1kg"(FALSE ("Sugar  1kg")) -> ()
    n243 = local write "Turmeric Powder 50g"(FALSE ("Turmeric Powder 50g")) -> ()
    n244 = local write "Carrot"(FALSE ("Carrot")) -> ()
    n245 = local write "Cabege"(FALSE ("Cabege")) -> ()
    n246 = local write "Curry Powder 100g"(FALSE ("Curry Powder 100g")) -> ()
    n247 = local write "Rise 5Kg"(FALSE ("Rise 5Kg")) -> ()
    n248 = local write "Coconut Oil 1L"(FALSE ("Coconut Oil 1L")) -> ()
    n249 = local write "Tea 100g"(FALSE ("Tea 100g")) -> ()
    n250 = local write "Salt 400g"(FALSE ("Salt 400g")) -> ()
    n251 = local write "Discount percentage"("0" ("Discount percentage")) -> ()
  }
